vi "FlexMag - 23-03-2023.vi"() -> ()   [LabVIEW 2018] (continued)
                n23229 = local read "L rf power step 1"() -> (w27290:string)
                n23230 = local read "L rf power step 7"() -> (w27302:string)
                n23231 = local read "L rf power step 2"() -> (w27246:string)
                n23232 = local read "L rf power step 4"() -> (w27241:string)
                n23233 = local read "L rf power step 2"() -> (w27289:string)
                n23234 = local read "L rf power step 4"() -> (w27294:string)
                n23235 = local read "L rf power step 3"() -> (w27242:string)
                n23236 = local read "L rf power step 5"() -> (w27228:string)
                n23237 = local read "L rf power step 6"() -> (w27234:string)
                n23238 = local read "L rf power step 3"() -> (w27293:string)
                n23239 = local read "L rf power step 5"() -> (w27307:string)
                n23240 = local read "L rf power step 6"() -> (w27301:string)
                n23241 = Decimal String To Number(string=w27231) -> (number=w27230:i32)  [unwired: 2 in, 1 out]
                n23242 = Decimal String To Number(string=w27304) -> (number=w27305:i32)  [unwired: 2 in, 1 out]
                n23243 = Decimal String To Number(string=w27238) -> (number=w27239:i32)  [unwired: 2 in, 1 out]
                n23244 = Decimal String To Number(string=w27297) -> (number=w27296:i32)  [unwired: 2 in, 1 out]
                n23245 = Decimal String To Number(string=w27237) -> (number=w27236:i32)  [unwired: 2 in, 1 out]
                n23246 = Decimal String To Number(string=w27298) -> (number=w27299:i32)  [unwired: 2 in, 1 out]
                n23247 = Decimal String To Number(string=w27245) -> (number=w27244:i32)  [unwired: 2 in, 1 out]
                n23248 = Decimal String To Number(string=w27233) -> (number=w27232:i32)  [unwired: 2 in, 1 out]
                n23249 = Decimal String To Number(string=w27290) -> (number=w27291:i32)  [unwired: 2 in, 1 out]
                n23250 = Decimal String To Number(string=w27302) -> (number=w27303:i32)  [unwired: 2 in, 1 out]
                n23251 = Decimal String To Number(string=w27246) -> (number=w27247:i32)  [unwired: 2 in, 1 out]
                n23252 = Decimal String To Number(string=w27241) -> (number=w27240:i32)  [unwired: 2 in, 1 out]
                n23253 = Decimal String To Number(string=w27289) -> (number=w27288:i32)  [unwired: 2 in, 1 out]
                n23254 = Decimal String To Number(string=w27294) -> (number=w27295:i32)  [unwired: 2 in, 1 out]
                n23255 = Decimal String To Number(string=w27242) -> (number=w27243:i32)  [unwired: 2 in, 1 out]
                n23256 = Decimal String To Number(string=w27228) -> (number=w27229:i32)  [unwired: 2 in, 1 out]
                n23257 = Decimal String To Number(string=w27234) -> (number=w27235:i32)  [unwired: 2 in, 1 out]
                n23258 = Decimal String To Number(string=w27293) -> (number=w27292:i32)  [unwired: 2 in, 1 out]
                n23259 = Decimal String To Number(string=w27307) -> (number=w27306:i32)  [unwired: 2 in, 1 out]
                n23260 = Decimal String To Number(string=w27301) -> (number=w27300:i32)  [unwired: 2 in, 1 out]
                n23261 = local write "R rf step power 10"(w27230) -> ()
                n23262 = local write "R rf step power 10"(w27305) -> ()
                n23263 = local write "R rf step power 9"(w27239) -> ()
                n23264 = local write "R rf step power 9"(w27296) -> ()
                n23265 = local write "R rf step power 8"(w27236) -> ()
                n23266 = local write "R rf step power 8"(w27299) -> ()
                n23267 = local write "R rf step power 1"(w27244) -> ()
                n23268 = local write "R rf step power 7"(w27232) -> ()
                n23269 = local write "R rf step power 1"(w27291) -> ()
                n23270 = local write "R rf step power 7"(w27303) -> ()
                n23271 = local write "R rf step power 2"(w27247) -> ()
                n23272 = local write "R rf step power 4"(w27240) -> ()
                n23273 = local write "R rf step power 2"(w27288) -> ()
                n23274 = local write "R rf step power 4"(w27295) -> ()
                n23275 = local write "R rf step power 3"(w27243) -> ()
                n23276 = local write "R rf step power 5"(w27229) -> ()
                n23277 = local write "R rf step power 6"(w27235) -> ()
                n23278 = local write "R rf step power 3"(w27292) -> ()
                n23279 = local write "R rf step power 5"(w27306) -> ()
                n23280 = local write "R rf step power 6"(w27300) -> ()
                n23281 = local read "L rf length step 1"() -> (w27210:string)
                n23282 = local read "L rf length step 10"() -> (w27224:string)
                n23283 = local read "L rf length step 7"() -> (w27222:string)
                n23284 = local read "L rf length step 1"() -> (w27326:string)
                n23285 = local read "L rf length step 10"() -> (w27312:string)
                n23286 = local read "L rf length step 2"() -> (w27209:string)
                n23287 = local read "L rf length step 4"() -> (w27214:string)
                n23288 = local read "L rf length step 7"() -> (w27314:string)
                n23289 = local read "L rf length step 9"() -> (w27217:string)
                n23290 = local read "L rf length step 2"() -> (w27327:string)
                n23291 = local read "L rf length step 4"() -> (w27322:string)
                n23292 = local read "L rf length step 3"() -> (w27213:string)
                n23293 = local read "L rf length step 5"() -> (w27227:string)
                n23294 = local read "L rf length step 6"() -> (w27221:string)
                n23295 = local read "L rf length step 8"() -> (w27218:string)
                n23296 = local read "L rf length step 9"() -> (w27319:string)
                n23297 = local read "L rf length step 3"() -> (w27323:string)
                n23298 = local read "L rf length step 5"() -> (w27309:string)
                n23299 = local read "L rf length step 6"() -> (w27315:string)
                n23300 = local read "L rf length step 8"() -> (w27318:string)
                n23301 = Decimal String To Number(string=w27210) -> (number=w27211:i32)  [unwired: 2 in, 1 out]
                n23302 = Decimal String To Number(string=w27222) -> (number=w27223:i32)  [unwired: 2 in, 1 out]
                n23303 = Decimal String To Number(string=w27326) -> (number=w27325:i32)  [unwired: 2 in, 1 out]
                n23304 = Decimal String To Number(string=w27209) -> (number=w27208:i32)  [unwired: 2 in, 1 out]
                n23305 = Decimal String To Number(string=w27214) -> (number=w27215:i32)  [unwired: 2 in, 1 out]
                n23306 = Decimal String To Number(string=w27314) -> (number=w27313:i32)  [unwired: 2 in, 1 out]
                n23307 = Decimal String To Number(string=w27217) -> (number=w27216:i32)  [unwired: 2 in, 1 out]
                n23308 = Decimal String To Number(string=w27224) -> (number=w27225:i32)  [unwired: 2 in, 1 out]
                n23309 = Decimal String To Number(string=w27327) -> (number=w27328:i32)  [unwired: 2 in, 1 out]
                n23310 = Decimal String To Number(string=w27322) -> (number=w27321:i32)  [unwired: 2 in, 1 out]
                n23311 = Decimal String To Number(string=w27213) -> (number=w27212:i32)  [unwired: 2 in, 1 out]
                n23312 = Decimal String To Number(string=w27227) -> (number=w27226:i32)  [unwired: 2 in, 1 out]
                n23313 = Decimal String To Number(string=w27221) -> (number=w27220:i32)  [unwired: 2 in, 1 out]
                n23314 = Decimal String To Number(string=w27218) -> (number=w27219:i32)  [unwired: 2 in, 1 out]
                n23315 = Decimal String To Number(string=w27319) -> (number=w27320:i32)  [unwired: 2 in, 1 out]
                n23316 = Decimal String To Number(string=w27312) -> (number=w27311:i32)  [unwired: 2 in, 1 out]
                n23317 = Decimal String To Number(string=w27323) -> (number=w27324:i32)  [unwired: 2 in, 1 out]
                n23318 = Decimal String To Number(string=w27309) -> (number=w27310:i32)  [unwired: 2 in, 1 out]
                n23319 = Decimal String To Number(string=w27315) -> (number=w27316:i32)  [unwired: 2 in, 1 out]
                n23320 = Decimal String To Number(string=w27318) -> (number=w27317:i32)  [unwired: 2 in, 1 out]
                n23321 = local write "R rf step length 1"(w27211) -> ()
                n23322 = local write "R rf step length 10"(w27225) -> ()
                n23323 = local write "R rf step length 7"(w27223) -> ()
                n23324 = local write "R rf step length 1"(w27325) -> ()
                n23325 = local write "R rf step length 10"(w27311) -> ()
                n23326 = local write "R rf step length 2"(w27208) -> ()
                n23327 = local write "R rf step length 4"(w27215) -> ()
                n23328 = local write "R rf step length 7"(w27313) -> ()
                n23329 = local write "R rf step length 9"(w27216) -> ()
                n23330 = local write "R rf step length 2"(w27328) -> ()
                n23331 = local write "R rf step length 4"(w27321) -> ()
                n23332 = local write "R rf step length 3"(w27212) -> ()
                n23333 = local write "R rf step length 5"(w27226) -> ()
                n23334 = local write "R rf step length 6"(w27220) -> ()
                n23335 = local write "R rf step length 8"(w27219) -> ()
                n23336 = local write "R rf step length 9"(w27320) -> ()
                n23337 = local write "R rf step length 3"(w27324) -> ()
                n23338 = local write "R rf step length 5"(w27310) -> ()
                n23339 = local write "R rf step length 6"(w27316) -> ()
                n23340 = local write "R rf step length 8"(w27317) -> ()
              }
            }
            n23341 = local read "L chamber selection"() -> (w27180:string)
            n23342 = local read "L recipe selection"() -> (w27205:string)
            n23343 = local read "L web selection"() -> (w27201:string)
            n23344 = Equal?(x=w27180, y="III" ("L single process")) -> (x = y?=w27178:bool)
            n23345 = local read "L recipe name"() -> (w27207:string)
            n23346 = Equal?(x=w27184, y="Microwave" ("L single process")) -> (x = y?=w27182:bool)
            n23347 = local read "L sbs name"() -> (w27206:string)
            n23348 = case shown="True" w27182 {
              tunnel: [w27371 enum32{"microwave", "dcsputter", "rfsputter"}."microwave" ("single process selection")] -> w27181
              frame False {
                n23349 = local read "L single process type selection"() -> (w27373:string)
                n23350 = Equal?(x=w27373, y="RF Sputter" ("L single process")) -> (x = y?=w27372:bool)
                n23351 = case shown="False" w27372 {
                  tunnel: [enum32{"microwave", "dcsputter", "rfsputter"}."dcsputter" ("single process selection") enum32{"microwave", "dcsputter", "rfsputter"}."rfsputter" ("single process selection")] -> w27371
                  frame False {
                  }
                  frame True {
                  }
                }
              }
              frame True {
              }
            }
            n23352 = case shown="False" w27178 {
              tunnel: [enum32{"chamber II", "chamber III"}."chamber II" ("DC Sputter Chamber Selection") enum32{"chamber II", "chamber III"}."chamber III" ("DC Sputter Chamber Selection")] -> w27177
              frame False {
              }
              frame True {
              }
            }
            n23353 = Equal?(x=w27201, y="Web") -> (x = y?=w27199:bool)
            n23354 = Equal?(x=w27205, y="Single Recipe") -> (x = y?=w27203:bool)
            n23355 = local write "R Substrate Material"(w27206) -> ()
            n23356 = case shown="True" w27203 {
              tunnel: [w27380 w27381] -> w27202
              frame False {
                w27380 = u16 1 items=["single recipe", "multilayer recipe"] ("Recipe Selection")
              }
              frame True {
                w27381 = u16 0 items=["single recipe", "multilayer recipe"] ("Recipe Selection")
              }
            }
            n23357 = case shown="False" w27199 {
              tunnel: [w27378 w27379] -> w27198
              frame False {
                w27378 = u16 1 items=["web", "other"] ("Web Selection")
              }
              frame True {
                w27379 = u16 0 items=["web", "other"] ("Web Selection")
              }
            }
            n23358 = local write "R Recipe Name"(w27207) -> ()
            n23359 = local write "R DC Sputter Chamber Selection"(w27177) -> ()
            n23360 = local write "R Recipe Selection"(w27202) -> ()
            n23361 = local write "R Web Selection"(w27198) -> ()
            n23362 = Wait (ms)(milliseconds to wait=u32 500) -> ()  [unwired: 1 out]
            n23363 = local write "R single process selection"(w27181) -> ()
            n23364 = local read "L left init diamater"() -> (w27196:string)
            n23365 = local read "L core diamater"() -> (w27197:string)
            n23366 = local read "L web thickness"() -> (w27191:string)
            n23367 = local read "L tension  value"() -> (w27187:string)
            n23368 = local read "L web speed"() -> (w27190:string)
            n23369 = local read "L pressure"() -> (w27173:string)
            n23370 = local read "L argon flow"() -> (w27171:string)
            n23371 = Decimal String To Number(string=w27197) -> (number=w27195:i32)  [unwired: 2 in, 1 out]
            n23372 = Decimal String To Number(string=w27191) -> (number=w27192:i32)  [unwired: 2 in, 1 out]
            n23373 = Decimal String To Number(string=w27187) -> (number=w27188:i32)  [unwired: 2 in, 1 out]
            n23374 = Decimal String To Number(string=w27190) -> (number=w27189:i32)  [unwired: 2 in, 1 out]
            n23375 = Fract/Exp String To Number(use system decimal point (T)=FALSE, string=w27196) -> (number=w27194:dbl)  [unwired: 2 in, 1 out]
            n23376 = Fract/Exp String To Number(use system decimal point (T)=FALSE, string=w27173) -> (number=w27174:dbl)  [unwired: 2 in, 1 out]
            n23377 = Decimal String To Number(string=w27171) -> (number=w27172:i32)  [unwired: 2 in, 1 out]
            n23378 = local write "R left initial diameter"(w27194) -> ()
            n23379 = local write "R core diameter"(w27195) -> ()
            n23380 = local write "R web thickness"(w27192) -> ()
            n23381 = local write "R tension value"(w27188) -> ()
            n23382 = local write "R Pressure set mbar"(w27174) -> ()
            n23383 = local write "R web speed"(w27189) -> ()
            n23384 = local write "R Ar set sccm"(w27172) -> ()
            n23385 = local read "L microwave power"() -> (w27185:string)
            n23386 = local read "L dc step numbers"() -> (w27169:string)
            n23387 = local read "L rf step numbers"() -> (w27170:string)
            n23388 = Decimal String To Number(string=w27185) -> (number=w27186:i32)  [unwired: 2 in, 1 out]
            n23389 = Decimal String To Number(string=w27169) -> (number=w27168:i32)  [unwired: 2 in, 1 out]
            n23390 = Decimal String To Number(string=w27170) -> (number=w27167:i32)  [unwired: 2 in, 1 out]
            n23391 = local write "R power microwave"(w27186) -> ()
            n23392 = local write "R RF number steps"(w27167) -> ()
            n23393 = local write "R DC number steps"(w27168) -> ()
          }
          frame #2 {
            n23394 = local write "load recipe from path"(FALSE ("load recipe from path")) -> ()
          }
        }
      }
    }
  }
  n23395 = while {
    stop <- FALSE stop-if-true
    n23396 = stacked-sequence {
      frame #0 {
        n23397 = local read "dcps on safety"() -> (w27388:bool)
        n23398 = local read "Dcps_is_on"() -> (w27389:bool)
        n23399 = Implies(1:w27388, 2:w27389) -> (0:w27390:bool)
        n23400 = feedback #347() -> (w27392:bool)  [unwired: 1 in]
        n23401 = Not(x=w27390) -> (.not. x?=w27391:bool)
        n23402 = case shown="True" w27391 {
          tunnel: w27392 -> [_ w27398]
          tunnel: [TRUE FALSE] -> w27387
          tunnel: [FALSE w27399] -> w27386
          frame False {
          }
          frame True {
            n23403 = call "Elapsed Time190"("Reset"=w27398) -> ("Elapsed Time (s)"=w27401:dbl)  [unwired: 11 in, 7 out]
            n23404 = Greater Or Equal?(x=w27401, y=8.0) -> (x >= y?=w27399:bool)
          }
        }
        n23405 = feedback-in #347(w27387) -> ()
        n23406 = case shown="True" w27386 {
          tunnel: [FALSE TRUE] -> w27385
          frame False {
          }
          frame True {
            n23407 = local write "Warning Message"("Problem with DC Power Supply !" ("Warning Message")) -> ()
          }
        }
        n23408 = local write "Dc_auto_off"(w27385) -> ()
      }
      frame #1 {
        n23409 = local read "chvbv1 open safety"() -> (w27441:bool)
        n23410 = local read "plvbv1 open safety"() -> (w27438:bool)
        n23411 = local read "bgbv1 open safety"() -> (w27427:bool)
        n23412 = local read "tpbv1 open safety"() -> (w27452:bool)
        n23413 = local read "sov1 open safety"() -> (w27417:bool)
        n23414 = local read "cc1 open safety"() -> (w27424:bool)
        n23415 = local read "mp1 start safety"() -> (w27466:bool)
        n23416 = local read "CH1_CH_VBV_DI"() -> (w27440:bool)
        n23417 = local read "CH1_PL_VBV_DI"() -> (w27439:bool)
        n23418 = local read "CH1_SoV_Ar_DI"() -> (w27418:bool)
        n23419 = local read "tp1 start safety"() -> (w27455:bool)
        n23420 = local read "CH1_BG_BV_DI"() -> (w27426:bool)
        n23421 = local read "CH1_TP_BV_DI"() -> (w27453:bool)
        n23422 = local read "CH1_CC_DI"() -> (w27425:bool)
        n23423 = local read "CH1_MP_DI"() -> (w27467:bool)
        n23424 = local read "ch1_tp_gui"() -> (w27454:bool)
        n23425 = Implies(1:w27466, 2:w27467) -> (0:w27465:bool)
        n23426 = Implies(1:w27455, 2:w27454) -> (0:w27456:bool)
        n23427 = Implies(1:w27452, 2:w27453) -> (0:w27451:bool)
        n23428 = Implies(1:w27441, 2:w27440) -> (0:w27442:bool)
        n23429 = Implies(1:w27438, 2:w27439) -> (0:w27437:bool)
        n23430 = Implies(1:w27424, 2:w27425) -> (0:w27423:bool)
        n23431 = Implies(1:w27427, 2:w27426) -> (0:w27428:bool)
        n23432 = Implies(1:w27417, 2:w27418) -> (0:w27416:bool)
        n23433 = feedback #348() -> (w27463:bool)  [unwired: 1 in]
        n23434 = feedback #349() -> (w27458:bool)  [unwired: 1 in]
        n23435 = feedback #350() -> (w27449:bool)  [unwired: 1 in]
        n23436 = feedback #351() -> (w27444:bool)  [unwired: 1 in]
        n23437 = feedback #352() -> (w27435:bool)  [unwired: 1 in]
        n23438 = feedback #353() -> (w27421:bool)  [unwired: 1 in]
        n23439 = feedback #354() -> (w27430:bool)  [unwired: 1 in]
        n23440 = feedback #355() -> (w27414:bool)  [unwired: 1 in]
        n23441 = Not(x=w27465) -> (.not. x?=w27464:bool)
        n23442 = Not(x=w27456) -> (.not. x?=w27457:bool)
        n23443 = Not(x=w27451) -> (.not. x?=w27450:bool)
        n23444 = Not(x=w27442) -> (.not. x?=w27443:bool)
        n23445 = Not(x=w27437) -> (.not. x?=w27436:bool)
        n23446 = Not(x=w27423) -> (.not. x?=w27422:bool)
        n23447 = Not(x=w27428) -> (.not. x?=w27429:bool)
        n23448 = Not(x=w27416) -> (.not. x?=w27415:bool)
        n23449 = case shown="True" w27464 {
          tunnel: w27463 -> [_ w27544]
          tunnel: [TRUE FALSE] -> w27462
          tunnel: [FALSE w27545] -> w27461
          frame False {
          }
          frame True {
            n23450 = call "Elapsed Time157"("Reset"=w27544) -> ("Elapsed Time (s)"=w27547:dbl)  [unwired: 11 in, 7 out]
            n23451 = Greater Or Equal?(x=w27547, y=8.0) -> (x >= y?=w27545:bool)
          }
        }
        n23452 = feedback-in #348(w27462) -> ()
        n23453 = case shown="True" w27457 {
          tunnel: w27458 -> [_ w27534]
          tunnel: [TRUE FALSE] -> w27459
          tunnel: [FALSE w27535] -> w27460
          frame False {
          }
          frame True {
            n23454 = call "Elapsed Time161"("Reset"=w27534) -> ("Elapsed Time (s)"=w27537:dbl)  [unwired: 11 in, 7 out]
            n23455 = Greater Or Equal?(x=w27537, y=8.0) -> (x >= y?=w27535:bool)
          }
        }
        n23456 = feedback-in #349(w27459) -> ()
        n23457 = case shown="True" w27450 {
          tunnel: w27449 -> [_ w27524]
          tunnel: [TRUE FALSE] -> w27448
          tunnel: [FALSE w27525] -> w27447
          frame False {
          }
          frame True {
            n23458 = call "Elapsed Time162"("Reset"=w27524) -> ("Elapsed Time (s)"=w27527:dbl)  [unwired: 11 in, 7 out]
            n23459 = Greater Or Equal?(x=w27527, y=8.0) -> (x >= y?=w27525:bool)
          }
        }
        n23460 = feedback-in #350(w27448) -> ()
        n23461 = case shown="True" w27443 {
          tunnel: w27444 -> [_ w27514]
          tunnel: [TRUE FALSE] -> w27445
          tunnel: [FALSE w27515] -> w27446
          frame False {
          }
          frame True {
            n23462 = call "Elapsed Time158"("Reset"=w27514) -> ("Elapsed Time (s)"=w27517:dbl)  [unwired: 11 in, 7 out]
            n23463 = Greater Or Equal?(x=w27517, y=8.0) -> (x >= y?=w27515:bool)
          }
        }
        n23464 = feedback-in #351(w27445) -> ()
        n23465 = case shown="True" w27436 {
          tunnel: w27435 -> [_ w27504]
          tunnel: [TRUE FALSE] -> w27434
          tunnel: [FALSE w27505] -> w27433
          frame False {
          }
          frame True {
            n23466 = call "Elapsed Time159"("Reset"=w27504) -> ("Elapsed Time (s)"=w27507:dbl)  [unwired: 11 in, 7 out]
            n23467 = Greater Or Equal?(x=w27507, y=8.0) -> (x >= y?=w27505:bool)
          }
        }
        n23468 = feedback-in #352(w27434) -> ()
        n23469 = case shown="True" w27422 {
          tunnel: w27421 -> [_ w27494]
          tunnel: [TRUE FALSE] -> w27420
          tunnel: [FALSE w27495] -> w27419
          frame False {
          }
          frame True {
            n23470 = call "Elapsed Time160"("Reset"=w27494) -> ("Elapsed Time (s)"=w27497:dbl)  [unwired: 11 in, 7 out]
            n23471 = Greater Or Equal?(x=w27497, y=8.0) -> (x >= y?=w27495:bool)
          }
        }
        n23472 = feedback-in #353(w27420) -> ()
        n23473 = case shown="True" w27429 {
          tunnel: w27430 -> [_ w27484]
          tunnel: [TRUE FALSE] -> w27431
          tunnel: [FALSE w27485] -> w27432
          frame False {
          }
          frame True {
            n23474 = call "Elapsed Time163"("Reset"=w27484) -> ("Elapsed Time (s)"=w27487:dbl)  [unwired: 11 in, 7 out]
            n23475 = Greater Or Equal?(x=w27487, y=8.0) -> (x >= y?=w27485:bool)
          }
        }
        n23476 = feedback-in #354(w27431) -> ()
        n23477 = case shown="True" w27415 {
          tunnel: w27414 -> [_ w27474]
          tunnel: [TRUE FALSE] -> w27413
          tunnel: [FALSE w27475] -> w27412
          frame False {
          }
          frame True {
            n23478 = call "Elapsed Time164"("Reset"=w27474) -> ("Elapsed Time (s)"=w27477:dbl)  [unwired: 11 in, 7 out]
            n23479 = Greater Or Equal?(x=w27477, y=8.0) -> (x >= y?=w27475:bool)
          }
        }
        n23480 = feedback-in #355(w27413) -> ()
        n23481 = case shown="True" w27461 {
          tunnel: [FALSE TRUE] -> w27411
          frame False {
          }
          frame True {
            n23482 = local write "Warning Message"("Problem with CH1 Mechanical Pump !\nCH1 ABORTED !" ("Warning Message")) -> ()
          }
        }
        n23483 = case shown="True" w27460 {
          tunnel: [FALSE TRUE] -> w27410
          frame False {
          }
          frame True {
            n23484 = local write "Warning Message"("Problem with CH1 Turbo Pump !\nCH1 ABORTED !" ("Warning Message")) -> ()
          }
        }
        n23485 = case shown="True" w27447 {
          tunnel: [FALSE TRUE] -> w27409
          frame False {
          }
          frame True {
            n23486 = local write "Warning Message"("Problem with CH1 Turbo Pump Block Valve !\nCH1 ABORTED !" ("Warning Message")) -> ()
          }
        }
        n23487 = case shown="True" w27446 {
          tunnel: [FALSE TRUE] -> w27408
          frame False {
          }
          frame True {
            n23488 = local write "Warning Message"("Problem with CH1 Chamber Vacuum Brake Valve !\nCH1 ABORTED !" ("Warning Message")) -> ()
          }
        }
        n23489 = case shown="True" w27433 {
          tunnel: [FALSE TRUE] -> w27407
          frame False {
          }
          frame True {
            n23490 = local write "Warning Message"("Problem with CH1 Pipeline Vacuum Brake Valve !\nCH1 ABORTED !" ("Warning Message")) -> ()
          }
        }
        n23491 = case shown="True" w27419 {
          tunnel: [FALSE TRUE] -> w27405
          frame False {
          }
          frame True {
            n23492 = local write "Warning Message"("Problem with CH1 Cold Cathode !\nCH1 CC has been closed !" ("Warning Message")) -> ()
          }
        }
        n23493 = case shown="True" w27432 {
          tunnel: [FALSE TRUE] -> w27404
          frame False {
          }
          frame True {
            n23494 = local write "Warning Message"("Problem with CH1 Baratron Gauge Block Valve !\nCH1 BG BV has been closed !" ("Warning Message")) -> ()
          }
        }
        n23495 = case shown="True" w27412 {
          tunnel: [FALSE TRUE] -> w27403
          frame False {
          }
          frame True {
            n23496 = local write "Warning Message"("Problem with CH1 Argon Shut of Valve !\nCH1 Ar SoV has been closed !" ("Warning Message")) -> ()
          }
        }
        n23497 = case shown="True" w27403 {
          frame False {
          }
          frame True {
            n23498 = local write "CH1_SoV_Ar_DO"(FALSE ("CH2_CC_DO")) -> ()
          }
        }
        n23499 = case shown="True" w27405 {
          frame False {
          }
          frame True {
            n23500 = local write "CH1_CC_DO"(FALSE ("CH2_CC_DO")) -> ()
          }
        }
        n23501 = case shown="True" w27404 {
          frame False {
          }
          frame True {
            n23502 = local write "CH1_BG_BV_DO"(FALSE ("CH2_CC_DO")) -> ()
          }
        }
        n23503 = Compound Arithmetic op=OR(w27411, w27410, w27409, w27408, w27407) -> (w27406:bool)
        n23504 = disable-structure shown="Disabled" {
          disable-tunnel: w27406 -> [w27468 _]
          frame Disabled {
            n23505 = local write "abort ch1"(w27468) -> ()
          }
          frame Enabled {
          }
        }
      }
      frame #2 {
        n23506 = local read "chvbv2 open safety"() -> (w27590:bool)
        n23507 = local read "plvbv2 open safety"() -> (w27587:bool)
        n23508 = local read "bgbv2 open safety"() -> (w27576:bool)
        n23509 = local read "tpbv2 open safety"() -> (w27601:bool)
        n23510 = local read "sov2 open safety"() -> (w27566:bool)
        n23511 = local read "cc2 open safety"() -> (w27573:bool)
        n23512 = local read "mp2 start safety"() -> (w27615:bool)
        n23513 = local read "CH2_CH_VBV_DI"() -> (w27589:bool)
        n23514 = local read "CH2_PL_VBV_DI"() -> (w27588:bool)
        n23515 = local read "CH2_SoV_Ar_DI"() -> (w27567:bool)
        n23516 = local read "tp2 start safety"() -> (w27604:bool)
        n23517 = local read "CH2_BG_BV_DI"() -> (w27575:bool)
        n23518 = local read "CH2_TP_BV_DI"() -> (w27602:bool)
        n23519 = local read "CH2_CC_DI"() -> (w27574:bool)
        n23520 = local read "CH2_MP_DI"() -> (w27616:bool)
        n23521 = local read "ch2_tp_gui"() -> (w27603:bool)
        n23522 = Implies(1:w27615, 2:w27616) -> (0:w27614:bool)
        n23523 = Implies(1:w27604, 2:w27603) -> (0:w27605:bool)
        n23524 = Implies(1:w27601, 2:w27602) -> (0:w27600:bool)
        n23525 = Implies(1:w27590, 2:w27589) -> (0:w27591:bool)
        n23526 = Implies(1:w27587, 2:w27588) -> (0:w27586:bool)
        n23527 = Implies(1:w27573, 2:w27574) -> (0:w27572:bool)
        n23528 = Implies(1:w27576, 2:w27575) -> (0:w27577:bool)
        n23529 = Implies(1:w27566, 2:w27567) -> (0:w27565:bool)
        n23530 = feedback #356() -> (w27612:bool)  [unwired: 1 in]
        n23531 = feedback #357() -> (w27607:bool)  [unwired: 1 in]
        n23532 = feedback #358() -> (w27598:bool)  [unwired: 1 in]
        n23533 = feedback #359() -> (w27593:bool)  [unwired: 1 in]
        n23534 = feedback #360() -> (w27584:bool)  [unwired: 1 in]
        n23535 = feedback #361() -> (w27570:bool)  [unwired: 1 in]
        n23536 = feedback #362() -> (w27579:bool)  [unwired: 1 in]
        n23537 = feedback #363() -> (w27563:bool)  [unwired: 1 in]
        n23538 = Not(x=w27614) -> (.not. x?=w27613:bool)
        n23539 = Not(x=w27605) -> (.not. x?=w27606:bool)
        n23540 = Not(x=w27600) -> (.not. x?=w27599:bool)
        n23541 = Not(x=w27591) -> (.not. x?=w27592:bool)
        n23542 = Not(x=w27586) -> (.not. x?=w27585:bool)
        n23543 = Not(x=w27572) -> (.not. x?=w27571:bool)
        n23544 = Not(x=w27577) -> (.not. x?=w27578:bool)
        n23545 = Not(x=w27565) -> (.not. x?=w27564:bool)
        n23546 = case shown="True" w27613 {
          tunnel: w27612 -> [_ w27693]
          tunnel: [TRUE FALSE] -> w27611
          tunnel: [FALSE w27694] -> w27610
          frame False {
          }
          frame True {
            n23547 = call "Elapsed Time165"("Reset"=w27693) -> ("Elapsed Time (s)"=w27696:dbl)  [unwired: 11 in, 7 out]
            n23548 = Greater Or Equal?(x=w27696, y=8.0) -> (x >= y?=w27694:bool)
          }
        }
        n23549 = feedback-in #356(w27611) -> ()
        n23550 = case shown="True" w27606 {
          tunnel: w27607 -> [_ w27683]
          tunnel: [TRUE FALSE] -> w27608
          tunnel: [FALSE w27684] -> w27609
          frame False {
          }
          frame True {
            n23551 = call "Elapsed Time166"("Reset"=w27683) -> ("Elapsed Time (s)"=w27686:dbl)  [unwired: 11 in, 7 out]
            n23552 = Greater Or Equal?(x=w27686, y=8.0) -> (x >= y?=w27684:bool)
          }
        }
        n23553 = feedback-in #357(w27608) -> ()
        n23554 = case shown="True" w27599 {
          tunnel: w27598 -> [_ w27673]
          tunnel: [TRUE FALSE] -> w27597
          tunnel: [FALSE w27674] -> w27596
          frame False {
          }
          frame True {
            n23555 = call "Elapsed Time167"("Reset"=w27673) -> ("Elapsed Time (s)"=w27676:dbl)  [unwired: 11 in, 7 out]
            n23556 = Greater Or Equal?(x=w27676, y=8.0) -> (x >= y?=w27674:bool)
          }
        }
        n23557 = feedback-in #358(w27597) -> ()
        n23558 = case shown="True" w27592 {
          tunnel: w27593 -> [_ w27663]
          tunnel: [TRUE FALSE] -> w27594
          tunnel: [FALSE w27664] -> w27595
          frame False {
          }
          frame True {
            n23559 = call "Elapsed Time168"("Reset"=w27663) -> ("Elapsed Time (s)"=w27666:dbl)  [unwired: 11 in, 7 out]
            n23560 = Greater Or Equal?(x=w27666, y=8.0) -> (x >= y?=w27664:bool)
          }
        }
        n23561 = feedback-in #359(w27594) -> ()
        n23562 = case shown="True" w27585 {
          tunnel: w27584 -> [_ w27653]
          tunnel: [TRUE FALSE] -> w27583
          tunnel: [FALSE w27654] -> w27582
          frame False {
          }
          frame True {
            n23563 = call "Elapsed Time169"("Reset"=w27653) -> ("Elapsed Time (s)"=w27656:dbl)  [unwired: 11 in, 7 out]
            n23564 = Greater Or Equal?(x=w27656, y=8.0) -> (x >= y?=w27654:bool)
          }
        }
        n23565 = feedback-in #360(w27583) -> ()
        n23566 = case shown="True" w27571 {
          tunnel: w27570 -> [_ w27643]
          tunnel: [TRUE FALSE] -> w27569
          tunnel: [FALSE w27644] -> w27568
          frame False {
          }
          frame True {
            n23567 = call "Elapsed Time170"("Reset"=w27643) -> ("Elapsed Time (s)"=w27646:dbl)  [unwired: 11 in, 7 out]
            n23568 = Greater Or Equal?(x=w27646, y=8.0) -> (x >= y?=w27644:bool)
          }
        }
        n23569 = feedback-in #361(w27569) -> ()
        n23570 = case shown="True" w27578 {
          tunnel: w27579 -> [_ w27633]
          tunnel: [TRUE FALSE] -> w27580
          tunnel: [FALSE w27634] -> w27581
          frame False {
          }
          frame True {
            n23571 = call "Elapsed Time171"("Reset"=w27633) -> ("Elapsed Time (s)"=w27636:dbl)  [unwired: 11 in, 7 out]
            n23572 = Greater Or Equal?(x=w27636, y=8.0) -> (x >= y?=w27634:bool)
          }
        }
        n23573 = feedback-in #362(w27580) -> ()
        n23574 = case shown="True" w27564 {
          tunnel: w27563 -> [_ w27623]
          tunnel: [TRUE FALSE] -> w27562
          tunnel: [FALSE w27624] -> w27561
          frame False {
          }
          frame True {
            n23575 = call "Elapsed Time172"("Reset"=w27623) -> ("Elapsed Time (s)"=w27626:dbl)  [unwired: 11 in, 7 out]
            n23576 = Greater Or Equal?(x=w27626, y=8.0) -> (x >= y?=w27624:bool)
          }
        }
        n23577 = feedback-in #363(w27562) -> ()
        n23578 = case shown="True" w27610 {
          tunnel: [FALSE TRUE] -> w27560
          frame False {
          }
          frame True {
            n23579 = local write "Warning Message"("Problem with CH2 Mechanical Pump !\nCH2 ABORTED !" ("Warning Message")) -> ()
          }
        }
        n23580 = case shown="True" w27609 {
          tunnel: [FALSE TRUE] -> w27559
          frame False {
          }
          frame True {
            n23581 = local write "Warning Message"("Problem with CH2 Turbo Pump !\nCH2 ABORTED !" ("Warning Message")) -> ()
          }
        }
        n23582 = case shown="True" w27596 {
          tunnel: [FALSE TRUE] -> w27558
          frame False {
          }
          frame True {
            n23583 = local write "Warning Message"("Problem with CH2 Turbo Pump Block Valve !\nCH2 ABORTED !" ("Warning Message")) -> ()
          }
        }
        n23584 = case shown="True" w27595 {
          tunnel: [FALSE TRUE] -> w27557
          frame False {
          }
          frame True {
            n23585 = local write "Warning Message"("Problem with CH2 Chamber Vacuum Brake Valve !\nCH2 ABORTED !" ("Warning Message")) -> ()
          }
        }
        n23586 = case shown="True" w27582 {
          tunnel: [FALSE TRUE] -> w27556
          frame False {
          }
          frame True {
            n23587 = local write "Warning Message"("Problem with CH2 Pipeline Vacuum Brake Valve !\nCH2 ABORTED !" ("Warning Message")) -> ()
          }
        }
        n23588 = case shown="True" w27568 {
          tunnel: [FALSE TRUE] -> w27554
          frame False {
          }
          frame True {
            n23589 = local write "Warning Message"("Problem with CH2 Cold Cathode !\nCH2 CC has been closed !" ("Warning Message")) -> ()
          }
        }
        n23590 = case shown="True" w27581 {
          tunnel: [FALSE TRUE] -> w27553
          frame False {
          }
          frame True {
            n23591 = local write "Warning Message"("Problem with CH2 Baratron Gauge Block Valve !\nCH2 BG BV has been closed !" ("Warning Message")) -> ()
          }
        }
        n23592 = case shown="True" w27561 {
          tunnel: [FALSE TRUE] -> w27552
          frame False {
          }
          frame True {
            n23593 = local write "Warning Message"("Problem with CH2 Argon Shut of Valve !\nCH2 Ar SoV has been closed !" ("Warning Message")) -> ()
          }
        }
        n23594 = case shown="True" w27552 {
          frame False {
          }
          frame True {
            n23595 = local write "CH2_SoV_Ar_DO"(FALSE ("CH2_CC_DO")) -> ()
          }
        }
        n23596 = case shown="True" w27554 {
          frame False {
          }
          frame True {
            n23597 = local write "CH2_CC_DO"(FALSE ("CH2_CC_DO")) -> ()
          }
        }
        n23598 = case shown="True" w27553 {
          frame False {
          }
          frame True {
            n23599 = local write "CH2_BG_BV_DO"(FALSE ("CH2_CC_DO")) -> ()
          }
        }
        n23600 = Compound Arithmetic op=OR(w27560, w27559, w27558, w27557, w27556) -> (w27555:bool)
        n23601 = disable-structure shown="Disabled" {
          disable-tunnel: w27555 -> [w27617 _]
          frame Disabled {
            n23602 = local write "abort ch2"(w27617) -> ()
          }
          frame Enabled {
          }
        }
      }
      frame #3 {
        n23603 = local read "chvbv3 open safety"() -> (w27739:bool)
        n23604 = local read "plvbv3 open safety"() -> (w27736:bool)
        n23605 = local read "bgbv3 open safety"() -> (w27725:bool)
        n23606 = local read "tpbv3 open safety"() -> (w27750:bool)
        n23607 = local read "sov3 open safety"() -> (w27715:bool)
        n23608 = local read "cc3 open safety"() -> (w27722:bool)
        n23609 = local read "CH3_SoV_Ar_DI"() -> (w27716:bool)
        n23610 = local read "mp3 start safety"() -> (w27764:bool)
        n23611 = local read "CH3_CH_VBV_DI"() -> (w27738:bool)
        n23612 = local read "CH3_PL_VBV_DI"() -> (w27737:bool)
        n23613 = local read "tp3 start safety"() -> (w27753:bool)
        n23614 = local read "CH3_BG_BV_DI"() -> (w27724:bool)
        n23615 = local read "CH3_TP_BV_DI"() -> (w27751:bool)
        n23616 = local read "CH3_CC_DI"() -> (w27723:bool)
        n23617 = local read "CH3_MP_DI"() -> (w27765:bool)
        n23618 = local read "ch3_tp_gui"() -> (w27752:bool)
        n23619 = Implies(1:w27764, 2:w27765) -> (0:w27763:bool)
        n23620 = Implies(1:w27753, 2:w27752) -> (0:w27754:bool)
        n23621 = Implies(1:w27750, 2:w27751) -> (0:w27749:bool)
        n23622 = Implies(1:w27739, 2:w27738) -> (0:w27740:bool)
        n23623 = Implies(1:w27736, 2:w27737) -> (0:w27735:bool)
        n23624 = Implies(1:w27722, 2:w27723) -> (0:w27721:bool)
        n23625 = Implies(1:w27725, 2:w27724) -> (0:w27726:bool)
        n23626 = Implies(1:w27715, 2:w27716) -> (0:w27714:bool)
        n23627 = feedback #364() -> (w27761:bool)  [unwired: 1 in]
        n23628 = feedback #365() -> (w27756:bool)  [unwired: 1 in]
        n23629 = feedback #366() -> (w27747:bool)  [unwired: 1 in]
        n23630 = feedback #367() -> (w27742:bool)  [unwired: 1 in]
        n23631 = feedback #368() -> (w27733:bool)  [unwired: 1 in]
        n23632 = feedback #369() -> (w27719:bool)  [unwired: 1 in]
        n23633 = feedback #370() -> (w27728:bool)  [unwired: 1 in]
        n23634 = feedback #371() -> (w27712:bool)  [unwired: 1 in]
        n23635 = Not(x=w27763) -> (.not. x?=w27762:bool)
        n23636 = Not(x=w27754) -> (.not. x?=w27755:bool)
        n23637 = Not(x=w27749) -> (.not. x?=w27748:bool)
        n23638 = Not(x=w27740) -> (.not. x?=w27741:bool)
        n23639 = Not(x=w27735) -> (.not. x?=w27734:bool)
        n23640 = Not(x=w27721) -> (.not. x?=w27720:bool)
        n23641 = Not(x=w27726) -> (.not. x?=w27727:bool)
        n23642 = Not(x=w27714) -> (.not. x?=w27713:bool)
        n23643 = case shown="True" w27762 {
          tunnel: w27761 -> [_ w27842]
          tunnel: [TRUE FALSE] -> w27760
          tunnel: [FALSE w27843] -> w27759
          frame False {
          }
          frame True {
            n23644 = call "Elapsed Time173"("Reset"=w27842) -> ("Elapsed Time (s)"=w27845:dbl)  [unwired: 11 in, 7 out]
            n23645 = Greater Or Equal?(x=w27845, y=8.0) -> (x >= y?=w27843:bool)
          }
        }
        n23646 = feedback-in #364(w27760) -> ()
        n23647 = case shown="True" w27755 {
          tunnel: w27756 -> [_ w27832]
          tunnel: [TRUE FALSE] -> w27757
          tunnel: [FALSE w27833] -> w27758
          frame False {
          }
          frame True {
            n23648 = call "Elapsed Time174"("Reset"=w27832) -> ("Elapsed Time (s)"=w27835:dbl)  [unwired: 11 in, 7 out]
            n23649 = Greater Or Equal?(x=w27835, y=8.0) -> (x >= y?=w27833:bool)
          }
        }
        n23650 = feedback-in #365(w27757) -> ()
        n23651 = case shown="True" w27748 {
          tunnel: w27747 -> [_ w27822]
          tunnel: [TRUE FALSE] -> w27746
          tunnel: [FALSE w27823] -> w27745
          frame False {
          }
          frame True {
            n23652 = call "Elapsed Time175"("Reset"=w27822) -> ("Elapsed Time (s)"=w27825:dbl)  [unwired: 11 in, 7 out]
            n23653 = Greater Or Equal?(x=w27825, y=8.0) -> (x >= y?=w27823:bool)
          }
        }
        n23654 = feedback-in #366(w27746) -> ()
        n23655 = case shown="True" w27741 {
          tunnel: w27742 -> [_ w27812]
          tunnel: [TRUE FALSE] -> w27743
          tunnel: [FALSE w27813] -> w27744
          frame False {
          }
          frame True {
            n23656 = call "Elapsed Time176"("Reset"=w27812) -> ("Elapsed Time (s)"=w27815:dbl)  [unwired: 11 in, 7 out]
            n23657 = Greater Or Equal?(x=w27815, y=8.0) -> (x >= y?=w27813:bool)
          }
        }
        n23658 = feedback-in #367(w27743) -> ()
        n23659 = case shown="True" w27734 {
          tunnel: w27733 -> [_ w27802]
          tunnel: [TRUE FALSE] -> w27732
          tunnel: [FALSE w27803] -> w27731
          frame False {
          }
          frame True {
            n23660 = call "Elapsed Time177"("Reset"=w27802) -> ("Elapsed Time (s)"=w27805:dbl)  [unwired: 11 in, 7 out]
            n23661 = Greater Or Equal?(x=w27805, y=8.0) -> (x >= y?=w27803:bool)
          }
        }
        n23662 = feedback-in #368(w27732) -> ()
        n23663 = case shown="True" w27720 {
          tunnel: w27719 -> [_ w27792]
          tunnel: [TRUE FALSE] -> w27718
          tunnel: [FALSE w27793] -> w27717
          frame False {
          }
          frame True {
            n23664 = call "Elapsed Time178"("Reset"=w27792) -> ("Elapsed Time (s)"=w27795:dbl)  [unwired: 11 in, 7 out]
            n23665 = Greater Or Equal?(x=w27795, y=8.0) -> (x >= y?=w27793:bool)
          }
        }
        n23666 = feedback-in #369(w27718) -> ()
        n23667 = case shown="True" w27727 {
          tunnel: w27728 -> [_ w27782]
          tunnel: [TRUE FALSE] -> w27729
          tunnel: [FALSE w27783] -> w27730
          frame False {
          }
          frame True {
            n23668 = call "Elapsed Time179"("Reset"=w27782) -> ("Elapsed Time (s)"=w27785:dbl)  [unwired: 11 in, 7 out]
            n23669 = Greater Or Equal?(x=w27785, y=8.0) -> (x >= y?=w27783:bool)
          }
        }
        n23670 = feedback-in #370(w27729) -> ()
        n23671 = case shown="True" w27713 {
          tunnel: w27712 -> [_ w27772]
          tunnel: [TRUE FALSE] -> w27711
          tunnel: [FALSE w27773] -> w27710
          frame False {
          }
          frame True {
            n23672 = call "Elapsed Time180"("Reset"=w27772) -> ("Elapsed Time (s)"=w27775:dbl)  [unwired: 11 in, 7 out]
            n23673 = Greater Or Equal?(x=w27775, y=8.0) -> (x >= y?=w27773:bool)
          }
        }
        n23674 = feedback-in #371(w27711) -> ()
        n23675 = case shown="True" w27759 {
          tunnel: [FALSE TRUE] -> w27709
          frame False {
          }
          frame True {
            n23676 = local write "Warning Message"("Problem with CH3 Mechanical Pump !\nCH3 ABORTED !" ("Warning Message")) -> ()
          }
        }
        n23677 = case shown="True" w27758 {
          tunnel: [FALSE TRUE] -> w27708
          frame False {
          }
          frame True {
            n23678 = local write "Warning Message"("Problem with CH3 Turbo Pump !\nCH3 ABORTED !" ("Warning Message")) -> ()
          }
        }
        n23679 = case shown="True" w27745 {
          tunnel: [FALSE TRUE] -> w27707
          frame False {
          }
          frame True {
            n23680 = local write "Warning Message"("Problem with CH3 Turbo Pump Block Valve !\nCH3 ABORTED !" ("Warning Message")) -> ()
          }
        }
        n23681 = case shown="True" w27744 {
          tunnel: [FALSE TRUE] -> w27706
          frame False {
          }
          frame True {
            n23682 = local write "Warning Message"("Problem with CH3 Chamber Vacuum Brake Valve !\nCH3 ABORTED !" ("Warning Message")) -> ()
          }
        }
        n23683 = case shown="True" w27731 {
          tunnel: [FALSE TRUE] -> w27705
          frame False {
          }
          frame True {
            n23684 = local write "Warning Message"("Problem with CH3 Pipeline Vacuum Brake Valve !\nCH3 ABORTED !" ("Warning Message")) -> ()
          }
        }
        n23685 = case shown="True" w27717 {
          tunnel: [FALSE TRUE] -> w27703
          frame False {
          }
          frame True {
            n23686 = local write "Warning Message"("Problem with CH3 Cold Cathode !\nCH3 CC has been closed !" ("Warning Message")) -> ()
          }
        }
        n23687 = case shown="True" w27730 {
          tunnel: [FALSE TRUE] -> w27702
          frame False {
          }
          frame True {
            n23688 = local write "Warning Message"("Problem with CH3 Baratron Gauge Block Valve !\nCH3 BG BV has been closed !" ("Warning Message")) -> ()
          }
        }
        n23689 = case shown="True" w27710 {
          tunnel: [FALSE TRUE] -> w27701
          frame False {
          }
          frame True {
            n23690 = local write "Warning Message"("Problem with CH3 Argon Shut of Valve !\nCH3 Ar SoV has been closed !" ("Warning Message")) -> ()
          }
        }
        n23691 = case shown="True" w27701 {
          frame False {
          }
          frame True {
            n23692 = local write "CH3_SoV_Ar_DO"(FALSE ("CH2_CC_DO")) -> ()
          }
        }
        n23693 = case shown="True" w27703 {
          frame False {
          }
          frame True {
            n23694 = local write "CH3_CC_DO"(FALSE ("CH2_CC_DO")) -> ()
          }
        }
        n23695 = case shown="True" w27702 {
          frame False {
          }
          frame True {
            n23696 = local write "CH3_BG_BV_DO"(FALSE ("CH2_CC_DO")) -> ()
          }
        }
        n23697 = Compound Arithmetic op=OR(w27709, w27708, w27707, w27706, w27705) -> (w27704:bool)
        n23698 = disable-structure shown="Disabled" {
          disable-tunnel: w27704 -> [w27766 _]
          frame Disabled {
            n23699 = local write "abort ch3"(w27766) -> ()
          }
          frame Enabled {
          }
        }
      }
      frame #4 {
        n23700 = local read "chvbv4 open safety"() -> (w27888:bool)
        n23701 = local read "plvbv4 open safety"() -> (w27885:bool)
        n23702 = local read "bgbv4 open safety"() -> (w27874:bool)
        n23703 = local read "tpbv4 open safety"() -> (w27899:bool)
        n23704 = local read "sov4 open safety"() -> (w27864:bool)
        n23705 = local read "cc4 open safety"() -> (w27871:bool)
        n23706 = local read "mp4 start safety"() -> (w27913:bool)
        n23707 = local read "CH4_CH_VBV_DI"() -> (w27887:bool)
        n23708 = local read "CH4_PL_VBV_DI"() -> (w27886:bool)
        n23709 = local read "CH4_SoV_Ar_DI"() -> (w27865:bool)
        n23710 = local read "tp4 start safety"() -> (w27902:bool)
        n23711 = local read "CH4_BG_BV_DI"() -> (w27873:bool)
        n23712 = local read "CH4_TP_BV_DI"() -> (w27900:bool)
        n23713 = local read "CH4_CC_DI"() -> (w27872:bool)
        n23714 = local read "CH4_MP_DI"() -> (w27914:bool)
        n23715 = local read "ch4_tp_gui"() -> (w27901:bool)
        n23716 = Implies(1:w27913, 2:w27914) -> (0:w27912:bool)
        n23717 = Implies(1:w27902, 2:w27901) -> (0:w27903:bool)
        n23718 = Implies(1:w27899, 2:w27900) -> (0:w27898:bool)
        n23719 = Implies(1:w27888, 2:w27887) -> (0:w27889:bool)
        n23720 = Implies(1:w27885, 2:w27886) -> (0:w27884:bool)
        n23721 = Implies(1:w27871, 2:w27872) -> (0:w27870:bool)
        n23722 = Implies(1:w27874, 2:w27873) -> (0:w27875:bool)
        n23723 = Implies(1:w27864, 2:w27865) -> (0:w27863:bool)
        n23724 = feedback #372() -> (w27910:bool)  [unwired: 1 in]
        n23725 = feedback #373() -> (w27905:bool)  [unwired: 1 in]
        n23726 = feedback #374() -> (w27896:bool)  [unwired: 1 in]
        n23727 = feedback #375() -> (w27891:bool)  [unwired: 1 in]
        n23728 = feedback #376() -> (w27882:bool)  [unwired: 1 in]
        n23729 = feedback #377() -> (w27868:bool)  [unwired: 1 in]
        n23730 = feedback #378() -> (w27877:bool)  [unwired: 1 in]
        n23731 = feedback #379() -> (w27861:bool)  [unwired: 1 in]
        n23732 = Not(x=w27912) -> (.not. x?=w27911:bool)
        n23733 = Not(x=w27903) -> (.not. x?=w27904:bool)
        n23734 = Not(x=w27898) -> (.not. x?=w27897:bool)
        n23735 = Not(x=w27889) -> (.not. x?=w27890:bool)
        n23736 = Not(x=w27884) -> (.not. x?=w27883:bool)
        n23737 = Not(x=w27870) -> (.not. x?=w27869:bool)
        n23738 = Not(x=w27875) -> (.not. x?=w27876:bool)
        n23739 = Not(x=w27863) -> (.not. x?=w27862:bool)
        n23740 = case shown="True" w27911 {
          tunnel: w27910 -> [_ w27991]
          tunnel: [TRUE FALSE] -> w27909
          tunnel: [FALSE w27992] -> w27908
          frame False {
          }
          frame True {
            n23741 = call "Elapsed Time181"("Reset"=w27991) -> ("Elapsed Time (s)"=w27994:dbl)  [unwired: 11 in, 7 out]
            n23742 = Greater Or Equal?(x=w27994, y=8.0) -> (x >= y?=w27992:bool)
          }
        }
        n23743 = feedback-in #372(w27909) -> ()
        n23744 = case shown="True" w27904 {
          tunnel: w27905 -> [_ w27981]
          tunnel: [TRUE FALSE] -> w27906
          tunnel: [FALSE w27982] -> w27907
          frame False {
          }
          frame True {
            n23745 = call "Elapsed Time182"("Reset"=w27981) -> ("Elapsed Time (s)"=w27984:dbl)  [unwired: 11 in, 7 out]
            n23746 = Greater Or Equal?(x=w27984, y=8.0) -> (x >= y?=w27982:bool)
          }
        }
        n23747 = feedback-in #373(w27906) -> ()
        n23748 = case shown="True" w27897 {
          tunnel: w27896 -> [_ w27971]
          tunnel: [TRUE FALSE] -> w27895
          tunnel: [FALSE w27972] -> w27894
          frame False {
          }
          frame True {
            n23749 = call "Elapsed Time183"("Reset"=w27971) -> ("Elapsed Time (s)"=w27974:dbl)  [unwired: 11 in, 7 out]
            n23750 = Greater Or Equal?(x=w27974, y=8.0) -> (x >= y?=w27972:bool)
          }
        }
        n23751 = feedback-in #374(w27895) -> ()
        n23752 = case shown="True" w27890 {
          tunnel: w27891 -> [_ w27961]
          tunnel: [TRUE FALSE] -> w27892
          tunnel: [FALSE w27962] -> w27893
          frame False {
          }
          frame True {
            n23753 = call "Elapsed Time184"("Reset"=w27961) -> ("Elapsed Time (s)"=w27964:dbl)  [unwired: 11 in, 7 out]
            n23754 = Greater Or Equal?(x=w27964, y=8.0) -> (x >= y?=w27962:bool)
          }
        }
        n23755 = feedback-in #375(w27892) -> ()
        n23756 = case shown="True" w27883 {
          tunnel: w27882 -> [_ w27951]
          tunnel: [TRUE FALSE] -> w27881
          tunnel: [FALSE w27952] -> w27880
          frame False {
          }
          frame True {
            n23757 = call "Elapsed Time185"("Reset"=w27951) -> ("Elapsed Time (s)"=w27954:dbl)  [unwired: 11 in, 7 out]
            n23758 = Greater Or Equal?(x=w27954, y=8.0) -> (x >= y?=w27952:bool)
          }
        }
        n23759 = feedback-in #376(w27881) -> ()
        n23760 = case shown="True" w27869 {
          tunnel: w27868 -> [_ w27941]
          tunnel: [TRUE FALSE] -> w27867
          tunnel: [FALSE w27942] -> w27866
          frame False {
          }
          frame True {
            n23761 = call "Elapsed Time186"("Reset"=w27941) -> ("Elapsed Time (s)"=w27944:dbl)  [unwired: 11 in, 7 out]
            n23762 = Greater Or Equal?(x=w27944, y=8.0) -> (x >= y?=w27942:bool)
          }
        }
        n23763 = feedback-in #377(w27867) -> ()
        n23764 = case shown="True" w27876 {
          tunnel: w27877 -> [_ w27931]
          tunnel: [TRUE FALSE] -> w27878
          tunnel: [FALSE w27932] -> w27879
          frame False {
          }
          frame True {
            n23765 = call "Elapsed Time187"("Reset"=w27931) -> ("Elapsed Time (s)"=w27934:dbl)  [unwired: 11 in, 7 out]
            n23766 = Greater Or Equal?(x=w27934, y=8.0) -> (x >= y?=w27932:bool)
          }
        }
        n23767 = feedback-in #378(w27878) -> ()
        n23768 = case shown="True" w27862 {
          tunnel: w27861 -> [_ w27921]
          tunnel: [TRUE FALSE] -> w27860
          tunnel: [FALSE w27922] -> w27859
          frame False {
          }
          frame True {
            n23769 = call "Elapsed Time188"("Reset"=w27921) -> ("Elapsed Time (s)"=w27924:dbl)  [unwired: 11 in, 7 out]
            n23770 = Greater Or Equal?(x=w27924, y=8.0) -> (x >= y?=w27922:bool)
          }
        }
        n23771 = feedback-in #379(w27860) -> ()
        n23772 = case shown="True" w27908 {
          tunnel: [FALSE TRUE] -> w27858
          frame False {
          }
          frame True {
            n23773 = local write "Warning Message"("Problem with CH4 Mechanical Pump !\nCH4 ABORTED !" ("Warning Message")) -> ()
          }
        }
        n23774 = case shown="True" w27907 {
          tunnel: [FALSE TRUE] -> w27857
          frame False {
          }
          frame True {
            n23775 = local write "Warning Message"("Problem with CH4 Turbo Pump !\nCH4 ABORTED !" ("Warning Message")) -> ()
          }
        }
        n23776 = case shown="True" w27894 {
          tunnel: [FALSE TRUE] -> w27856
          frame False {
          }
          frame True {
            n23777 = local write "Warning Message"("Problem with CH4 Turbo Pump Block Valve !\nCH4 ABORTED !" ("Warning Message")) -> ()
          }
        }
        n23778 = case shown="True" w27893 {
          tunnel: [FALSE TRUE] -> w27855
          frame False {
          }
          frame True {
            n23779 = local write "Warning Message"("Problem with CH4 Chamber Vacuum Brake Valve !\nCH4 ABORTED !" ("Warning Message")) -> ()
          }
        }
        n23780 = case shown="True" w27880 {
          tunnel: [FALSE TRUE] -> w27854
          frame False {
          }
          frame True {
            n23781 = local write "Warning Message"("Problem with CH4 Pipeline Vacuum Brake Valve !\nCH4 ABORTED !" ("Warning Message")) -> ()
          }
        }
        n23782 = case shown="True" w27866 {
          tunnel: [FALSE TRUE] -> w27852
          frame False {
          }
          frame True {
            n23783 = local write "Warning Message"("Problem with CH4 Cold Cathode !\nCH4 CC has been closed !" ("Warning Message")) -> ()
          }
        }
        n23784 = case shown="True" w27879 {
          tunnel: [FALSE TRUE] -> w27851
          frame False {
          }
          frame True {
            n23785 = local write "Warning Message"("Problem with CH4 Baratron Gauge Block Valve !\nCH4 BG BV has been closed !" ("Warning Message")) -> ()
          }
        }
        n23786 = case shown="True" w27859 {
          tunnel: [FALSE TRUE] -> w27850
          frame False {
          }
          frame True {
            n23787 = local write "Warning Message"("Problem with CH4 Argon Shut of Valve !\nCH4 Ar SoV has been closed !" ("Warning Message")) -> ()
          }
        }
        n23788 = case shown="True" w27850 {
          frame False {
          }
          frame True {
            n23789 = local write "CH4_SoV_Ar_DO"(FALSE ("CH2_CC_DO")) -> ()
          }
        }
        n23790 = case shown="True" w27852 {
          frame False {
          }
          frame True {
            n23791 = local write "CH4_CC_DO"(FALSE ("CH2_CC_DO")) -> ()
          }
        }
        n23792 = case shown="True" w27851 {
          frame False {
          }
          frame True {
            n23793 = local write "CH4_BG_BV_DO"(FALSE ("CH2_CC_DO")) -> ()
          }
        }
        n23794 = Compound Arithmetic op=OR(w27858, w27857, w27856, w27855, w27854) -> (w27853:bool)
        n23795 = disable-structure shown="Disabled" {
          disable-tunnel: w27853 -> [w27915 _]
          frame Disabled {
            n23796 = local write "abort ch4"(w27915) -> ()
          }
          frame Enabled {
          }
        }
      }
    }
    n23797 = Wait Until Next ms Multiple(millisecond multiple=u32 300) -> ()  [unwired: 1 out]
  }
  "Description" <- "" ("String")
  "Warning Message" <- "" ("Warning Message")
  "System Status" <- "SEMI-AUTOMATIC MODE " ("String")
  "ch1_door_open" <- w31
  "ch2_door_open" <- w31
  "ch3_door_open" <- w31
  "ch4_door_open" <- w31
  "backroll stop cmd" <- w14
  "forroll stop cmd" <- w14
  "rolling direction gui" <- w1
